vi "ScanCameraFocus.vi"() -> ()   [LabVIEW 2016] (continued)
  out "Match score vs displacement":cluster{dbl[], sgl[]}(graph)={[-2.0, -1.9, -1.8, -1.7, -1.6, -1.5, -1.4, -1.2999999999999998, -1.2, -1.1, -1.0, -0.8999999999999999, -0.7999999999999998, -0.7, -0.5999999999999999, -0.5, -0.3999999999999999, -0.2999999999999998, -0.19999999999999996, -0.09999999999999987, 0.0, 0.10000000000000009, 0.20000000000000018, 0.30000000000000027, 0.40000000000000036, 0.5, 0.6000000000000001, 0.7000000000000002, 0.8000000000000003, 0.9000000000000004, 1.0, 1.1, 1.2000000000000002, 1.3000000000000003, 1.4000000000000004, 1.5, 1.6, 1.7000000000000002, 1.8000000000000003, 1.9000000000000004, 2.0, 2.1000000000000005, 2.2, 2.3, 2.4000000000000004, 2.5, 2.6000000000000005, 2.7, 2.8000000000000007, 2.9000000000000004, 3.0, 3.1000000000000005, 3.2, 3.3000000000000007, 3.4000000000000004, 3.5, 3.6000000000000005, 3.7, 3.8000000000000007, 3.9000000000000004, 4.0, 4.1000000000000005, 4.2, 4.300000000000001, 4.4, 4.5, 4.6000000000000005, 4.7, 4.800000000000001, 4.9, 5.0, 5.1000000000000005, 5.2, 5.300000000000001, 5.4, 5.5, 5.6000000000000005, 5.7, 5.800000000000001, 5.9, 6.0, 6.1, 6.200000000000001, 6.300000000000001, 6.4, 6.5, 6.6, 6.700000000000001, 6.800000000000001, 6.9, 7.0, 7.1, 7.200000000000001, 7.300000000000001, 7.4, 7.5, 7.600000000000001, 7.700000000000001, 7.800000000000001, 7.9, 8.0, 8.100000000000001, 8.200000000000001, 8.3, 8.4, 8.5, 8.600000000000001, 8.700000000000001, 8.8, 8.9, 9.0, 9.100000000000001, 9.200000000000001, 9.3, 9.4, 9.5, 9.600000000000001, 9.700000000000001, 9.8, 9.9, 10.0], [869.16, 870.1541, 871.39026, 872.55273, 873.6957, 875.25287, 876.31866, 877.9247, 879.2218, 880.4835, 881.8531, 883.09845, 884.34955, 886.17163, 887.5967, 888.8688, 890.27716, 892.02856, 893.73047, 895.31525, 896.9751, 898.5983, 900.21747, 902.1295, 904.04614, 905.8335, 907.88635, 910.31226, 912.42053, 914.553, 917.0437, 919.398, 921.9271, 924.781, 928.02673, 931.43286, 934.40283, 937.87115, 941.5338, 945.68744, 948.91864, 952.5989, 956.83673, 960.76074, 964.0517, 967.93036, 970.9311, 973.84906, 976.09045, 976.83105, 978.2025, 977.4351, 976.63086, 976.10803, 972.1438, 968.2719, 965.92584, 962.9048, 957.64667, 955.20544, 950.172, 946.14453, 940.74744, 938.06586, 934.0315, 930.2287, 926.7642, 923.40344, 920.183, 917.18445, 913.9989, 911.6928, 909.2186, 906.7086, 904.7015, 902.61487, 900.4853, 898.55743, 896.5968, 894.7702, 893.13806, 891.5336, 890.0522, 888.5804, 886.85406, 885.3486, 884.04974, 882.66174, 881.2819, 879.8848, 878.6075, 877.4188, 876.1414, 875.2497, 874.0843, 872.85974, 871.7597, 870.1826, 869.6278, 868.561, 867.4404, 866.34564, 865.29114, 864.1999, 863.2289, 862.2323, 861.2315, 859.92535, 859.2958, 858.47675, 857.529, 856.49744, 855.59875, 854.7043, 853.684, 852.79486, 851.9777, 851.04254, 849.966, 848.84424, 848.2957]}
  in  "Match position variation tolerance":sgl=0.25
  out "Z step":dbl=12.0
  out "Image":T1(plugin-control)
  in  "End Z [mm]":dbl=10.0
  in  "Stepsize [mm]":dbl=0.1
  out "Matches (pixel)":T2(array[cluster])=[{"Position"={"x"=1325.479, "y"=883.1293}, "Angle"=0.0, "Scale"=1.0, "Score"=848.2957, "Bounding Box"=[{"x"=657.979, "y"=123.62927}, {"x"=1992.979, "y"=123.62927}, {"x"=1992.979, "y"=1642.6293}, {"x"=657.979, "y"=1642.6293}, {"x"=657.979, "y"=123.62927}]}] {"Bounding Box"."y" format="%.2f"; "Bounding Box"."x" format="%.2f"; "Score" format="%.2f"; "Scale" format="%.2f"; "Angle" format="%.2f"; "Position"."y" format="%.2f"; "Position"."x" format="%.2f"}
  in  "Match parameters":T3={"Number of Matches Requested"=10, "Minimum Match Score"=500.0, "Angle Ranges"=[]}
  in  "Template File Path":path=path "E:/XYZstage+Camera_CollectedImages/12-14-2016/test_sub_highVoltageContact_-23,-32,3.png"
  in  "Axes Speeds [mm/s]":T4={"X Speed"=25.0, "Y Speed"=3.0, "Z Speed"=1.0}
  in  "Initial Location [mm]":T5={"Go to X"=-23.0, "Go to Y"=-32.0, "Go to Z"=-2.0}
  out "Intensity histogram":T6(graph)={"Starting Value"=0.0, "Incremental Value"=1.0, "Histogram"=[77, 310, 1440, 5160, 11707, 21949, 34592, 44040, 61522, 59090, 132881, 181990, 251107, 301599, 277254, 244606, 193626, 125059, 84284, 56323, 35192, 26906, 21597, 17679, 17225, 17011, 10413, 15370, 16520, 15123, 15770, 17568, 16628, 17646, 19451, 17637, 17348, 18783, 16992, 16866, 17857, 16113, 16184, 11662, 16245, 16158, 17494, 16810, 15916, 17260, 16124, 15958, 17021, 16112, 16129, 17034, 15913, 16079, 17096, 15953, 15989, 11536, 16913, 15935, 16847, 16721, 15742, 16537, 17175, 16274, 17105, 17194, 15815, 16580, 16529, 15639, 16024, 15564, 9392, 14100, 14721, 13396, 13560, 14372, 12856, 12836, 13406, 12347, 12091, 12742, 11182, 10888, 11469, 10124, 10025, 10448, 6173, 8856, 9105, 8444, 8061, 8191, 7480, 6963, 7369, 6809, 6453, 6776, 6032, 6067, 6070, 5643, 5289, 3648, 5223, 4907, 4879, 4890, 4361, 4271, 4386, 3978, 4210, 4169, 3975, 3980, 4099, 3655, 3916, 4001, 2490, 3768, 4223, 3979, 4160, 4854, 4741, 5001, 6083, 5999, 6306, 7546, 7880, 8054, 9986, 10168, 9929, 12164, 8022, 12068, 13981, 14724, 14558, 16354, 17360, 16932, 19805, 21358, 21427, 24182, 26203, 25943, 29027, 31067, 29801, 21290, 35655, 35089, 35112, 39088, 37066, 36357, 40319, 38884, 37565, 39954, 37330, 34710, 36959, 34631, 33043, 33818, 30568, 18483, 30035, 26196, 23730, 24039, 20585, 18657, 18863, 16639, 14661, 15185, 12656, 11329, 11618, 9913, 8893, 9157, 5125, 7505, 7274, 6773, 6163, 6256, 5732, 5131, 5344, 4838, 4514, 4667, 4285, 3942, 4133, 3749, 3539, 2267, 3278, 3064, 2952, 2996, 2796, 2575, 2515, 2270, 2133, 2192, 2033, 1877, 1935, 1770, 1663, 1726, 1601, 873, 1561, 1334, 1290, 1371, 1263, 1161, 1232, 1123, 1121, 1221, 1048, 928, 1086, 923, 859, 977, 529, 815, 851, 14587]}
  out "Moving":bool
  out "XYZ Stage Current Position":T7={"X [-750, 750 mm]"=-23.00047348022461, "Y [-150, 30 mm]"=-32.00033050537109, "Z [-50, 50 mm]"=10.000400000000003}
  out "Error report":errorcluster
  in  "Camera Name":refnum<k21>="cam0" caption="IMAQdx Session"
  # "ANALYSIS"
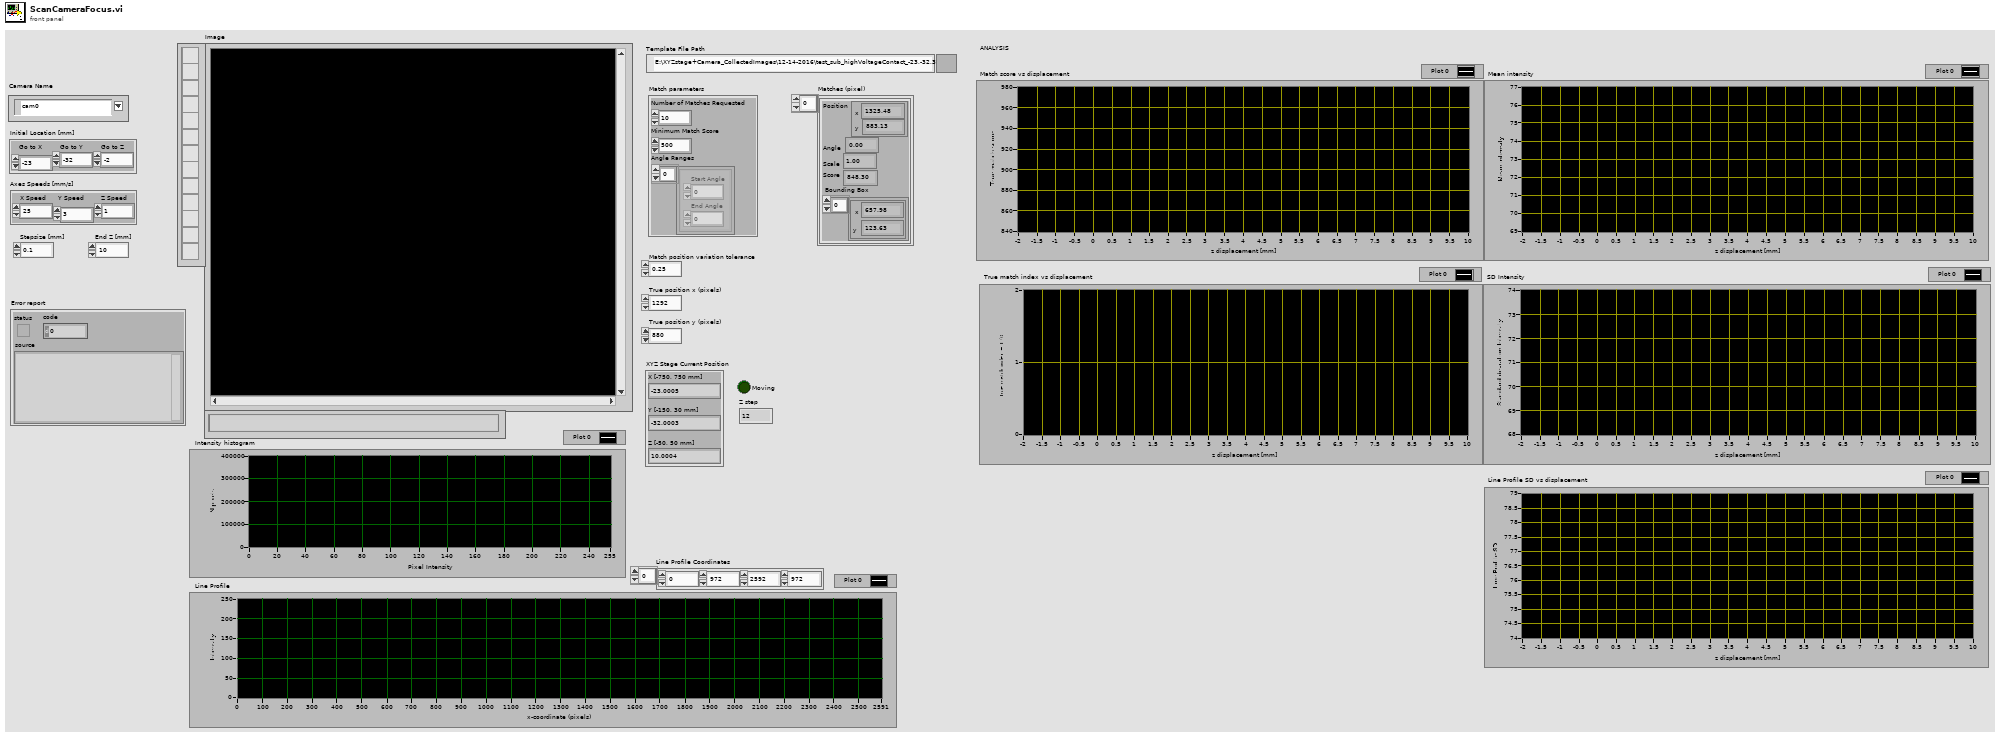
[diagram p1: front panel]
types:
  T1 = typedef "IMAQ Image.ctl" = refnum<image>
  T2 = cluster{"Position":cluster{"x":sgl, "y":sgl}, "Angle":sgl, "Scale":sgl, "Score":sgl, "Bounding Box":cluster{"x":sgl, "y":sgl}[]}[]
  T3 = cluster{"Number of Matches Requested":i32, "Minimum Match Score":sgl, "Angle Ranges":cluster{"Start Angle":sgl, "End Angle":sgl}[]}
  T4 = cluster{"X Speed":dbl, "Y Speed":dbl, "Z Speed":dbl}
  T5 = cluster{"Go to X":dbl, "Go to Y":dbl, "Go to Z":dbl}
  T6 = cluster{"Starting Value":sgl, "Incremental Value":sgl, "Histogram":u32[]}
  T7 = cluster{"X [-750, 750 mm]":dbl, "Y [-150, 30 mm]":dbl, "Z [-50, 50 mm]":dbl}
  T8 = typedef "Image Type" = u32
  T9 = typedef "IMAQdx.ctl" = refnum<k21>
  T10 = cluster{"Final X":dbl, "Final Y":dbl, "Final Z":dbl}
  T11 = cluster{"Min":sgl, "Max":sgl, "Mean":sgl, "Std Dev":sgl, "Count":i32}
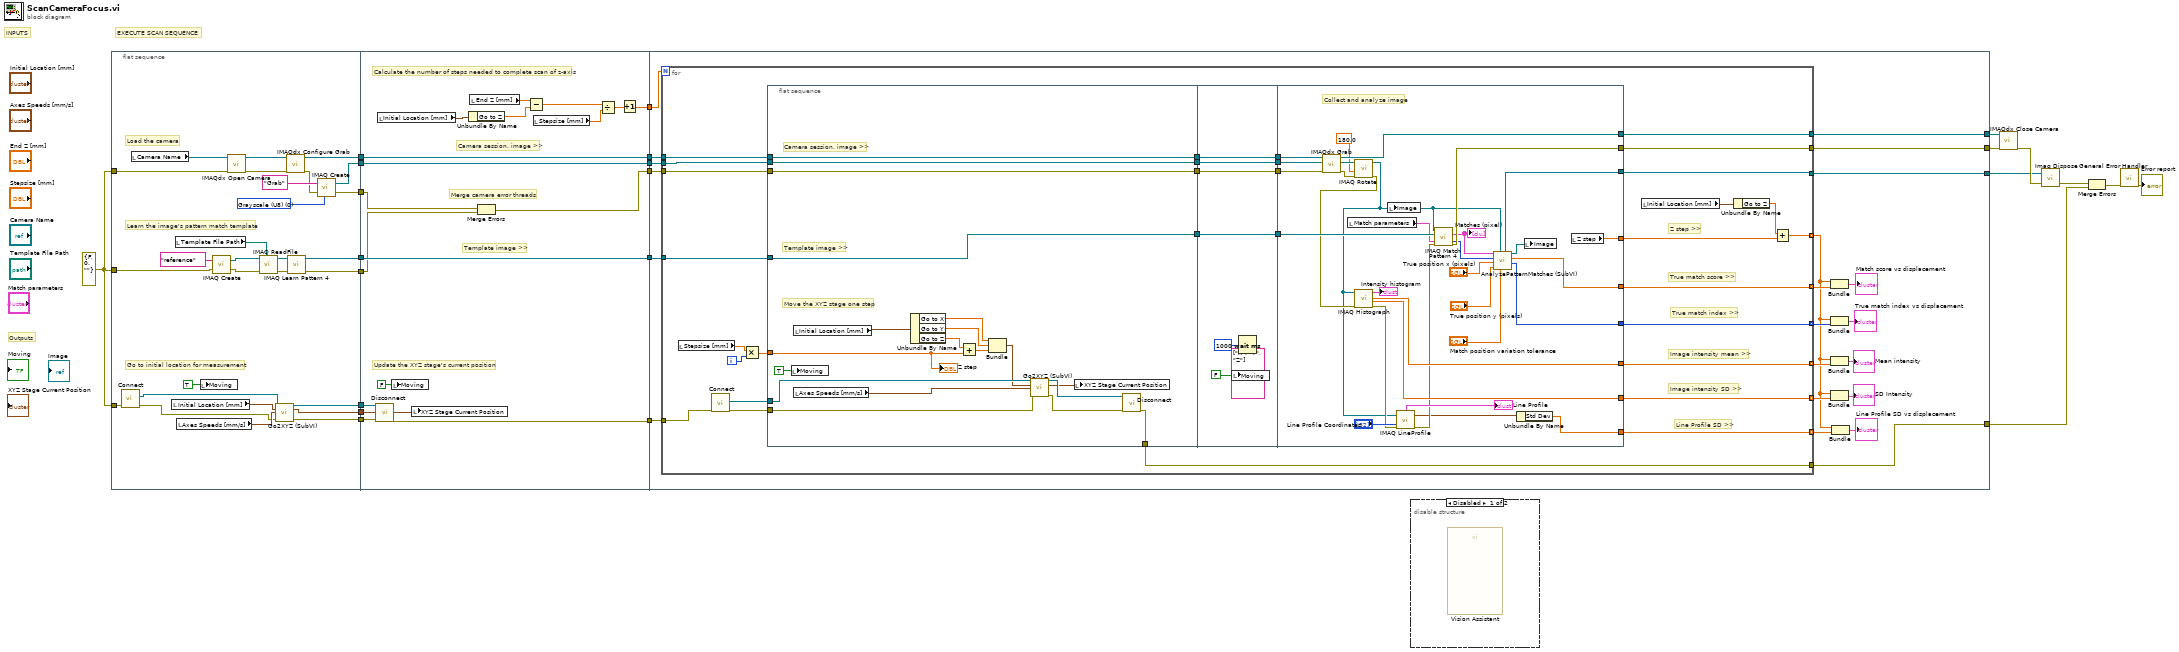
[diagram p0: block diagram]
diagram:
  w2 = errorcluster {"status"=FALSE, "code"=0, "source"=""} ("error in (no error)")
  # "EXECUTE SCAN SEQUENCE"
  # "Outputs"
  # "INPUTS"
  n1 = flat-sequence {
    tunnel: [w51] -> w19
    tunnel: [w50] -> w18
    tunnel: [w45] -> w17
    tunnel: [w34] -> w13
    tunnel: [w30] -> w12
    tunnel: [w29] -> w10
    tunnel: [w28] -> w7
    tunnel: [w27] -> w6
    tunnel: w2 -> [w26]
    tunnel: w2 -> [w25]
    tunnel: w2 -> [w24]
    tunnel: w19 -> [w64]
    tunnel: w18 -> [w63]
    tunnel: w17 -> [w68]
    tunnel: [w52] -> w16
    tunnel: [w62] -> w15
    tunnel: [w60] -> w14
    tunnel: w13 -> [w60]
    tunnel: w12 -> [w59]
    tunnel: [w59] -> w11
    tunnel: w10 -> [w57]
    tunnel: [w55] -> w9
    tunnel: [w58] -> w8
    tunnel: w7 -> [w58]
    tunnel: w6 -> [w56]
    tunnel: w16 -> [w82]
    tunnel: w15 -> [w90]
    tunnel: w14 -> [w89]
    tunnel: w11 -> [w88]
    tunnel: w9 -> [w87]
    tunnel: w8 -> [w86]
    tunnel: [w85] -> w5
    tunnel: [w84] -> w4
    tunnel: [w83] -> w3
    tunnel: [w75] -> w1
    frame #0 {
      w32 = T8 0 items=["Grayscale (U8)", "Grayscale (I16)", "Grayscale (SGL)", "Complex (CSG)", "RGB (U32)", "HSL (U32)", "RGB (U64)", "Grayscale (U16)"] ("Image Type")
      # "Learn the image's pattern match template"
      # "Load the camera"
      # "Go to initial location for measurement"
      n2 = call "Connect.vi"("error in (no error)"=w24) -> ("error out"=w44:errorcluster, "controller"=w46:refnum<k24>)  [unwired: 9 in]
      n3 = local read "Camera Name"() -> (w43:refnum<k21>)
      n4 = local read "Initial Location [mm]"() -> (w47:T5)
      n5 = local read "Template File Path"() -> (w40:path)
      n6 = local read "Axes Speeds [mm/s]"() -> (w48:T4)
      n7 = local write "Moving"(TRUE ("Moving")) -> ()
      n8 = call "IMAQ Create"("Image Name"="reference", "error in (no error)"=w26) -> ("New Image"=w39:T1, "error out"=w38:errorcluster)  [unwired: 3 in]
      n9 = call <vilib>:"IMAQdx Open Camera.vi"("error in"=w25, "Session In"=w43) -> ("error out"=w41:errorcluster, "Session Out"=w42:T9)  [unwired: 1 in, 7 out]
      n10 = call "IMAQ ReadFile"("File Path"=w40, "error in (no error)"=w38, "Image"=w39) -> ("error out"=w35:errorcluster, "Image Out"=w36:T1)  [unwired: 4 in, 3 out]
      n11 = call "Go2XYZ (SubVI).vi"(".NET Refnum in"=w46, "Go to Coordinates"=w47, "Axis Speeds"=w48, "error in (no error)"=w44) -> (".NET Refnum out"=w51:refnum<k24>, "Final Position"=w45:T10, "error out"=w50:errorcluster)  [unwired: 8 in, 1 out]
      n12 = call <vilib>:"IMAQdx Configure Grab.vi"("error in"=w41, "Session In"=w42) -> ("error out"=w31:errorcluster, "Session Out"=w34:T9)  [unwired: 8 out]
      n13 = call "IMAQ Learn Pattern 4"("error in (no error)"=w35, "Image"=w36) -> ("error out"=w27:errorcluster, "Template Image Out"=w28:T1)  [unwired: 7 in, 1 out]
      n14 = call "IMAQ Create"("Image Name"="Grab", "Image Type"=w32, "error in (no error)"=w31) -> ("New Image"=w30:T1, "error out"=w29:errorcluster)  [unwired: 1 in, 1 out]
    }
    frame #1 {
      # "Merge camera error threads"
      # "Camera session, image >>"
      # "Template image >>"
      # "Calculate the number of steps needed to complete scan of z-axis"
      # "Update the XYZ stage's current position"
      n15 = call "Disconnect.vi"("error in (no error)"=w63, "controller"=w64) -> ("error out"=w62:errorcluster)  [unwired: 9 in]
      n16 = local read "Initial Location [mm]"() -> (w67:T5)
      n17 = local write "Moving"(FALSE ("Moving")) -> ()
      n18 = local write "XYZ Stage Current Position"(w68) -> ()
      n19 = Unbundle By Name(w67) -> ("Go to Z"=w66:dbl)
      n20 = local read "End Z [mm]"() -> (w54:dbl)
      n21 = Merge Errors(w57, w56) -> (w55:errorcluster)
      n22 = Subtract(x=w54, y=w66) -> (x-y=w65:dbl)
      n23 = local read "Stepsize [mm]"() -> (w61:dbl)
      n24 = Divide(x=w65, y=w61) -> (x/y=w53:dbl)
      n25 = Increment(x=w53) -> (x+1=w52:dbl)
    }
    frame #2 {
      n26 = for {
        N: w82 -> [_]
        tunnel: w90 -> [w118]
        tunnel: w89 -> [w115]
        tunnel: w88 -> [w114]
        tunnel: w87 -> [w113]
        tunnel: w86 -> [w112]
        tunnel: [w111] -> w85
        tunnel: [w110] -> w84
        tunnel: [w109] -> w83
        tunnel: [w103] -> w71 mode=indexing
        tunnel: [w108] -> w81 mode=indexing
        tunnel: [w107] -> w80 mode=indexing
        tunnel: [w106] -> w79 mode=indexing
        tunnel: [w105] -> w75
        tunnel: [w92] -> w74 mode=indexing
        tunnel: [w91] -> w70 mode=indexing
        i -> [w120]
        (unwired) string[] ["X", "Y", "Z"] ("Axes Names")
        # "Line Profile SD >>"
        # "True match index >>"
        # "Image intensity SD >>"
        # "Image intensity mean >>"
        # "True match score >>"
        # "Z step >>"
        n27 = local read "Stepsize [mm]"() -> (w117:dbl)
        n28 = call "Connect.vi"("error in (no error)"=w118) -> ("error out"=w116:errorcluster, "controller"=w121:refnum<k24>)  [unwired: 9 in]
        n29 = Multiply(x=w117, y=w120) -> (x*y=w119:dbl)
        n30 = flat-sequence {
          tunnel: w121 -> [w140]
          tunnel: w116 -> [w139]
          tunnel: w119 -> [w134]
          tunnel: [w126] -> w100
          tunnel: w115 -> [w126]
          tunnel: w114 -> [w125]
          tunnel: [w125] -> w98
          tunnel: w113 -> [w124]
          tunnel: [w124] -> w96
          tunnel: [w123] -> w94
          tunnel: w112 -> [w123]
          tunnel: [w122] -> w110
          tunnel: w100 -> [w146]
          tunnel: [w146] -> w99
          tunnel: w98 -> [w145]
          tunnel: [w145] -> w97
          tunnel: w96 -> [w144]
          tunnel: [w144] -> w95
          tunnel: w94 -> [w143]
          tunnel: [w143] -> w93
          tunnel: w99 -> [w177]
          tunnel: w97 -> [w176]
          tunnel: w95 -> [w175]
          tunnel: w93 -> [w174]
          tunnel: [w166] -> w111
          tunnel: [w172] -> w109
          tunnel: [w170] -> w101
          tunnel: [w159] -> w108
          tunnel: [w169] -> w107
          tunnel: [w168] -> w106
          tunnel: [w167] -> w105
          tunnel: [w158] -> w92
          tunnel: [w148] -> w91
          frame #0 {
            # "Camera session, image >>"
            # "Template image >>"
            # "Move the XYZ stage one step"
            n31 = local write "Moving"(TRUE ("Moving")) -> ()
            n32 = local read "Initial Location [mm]"() -> (w136:T5)
            n33 = local read "Axes Speeds [mm/s]"() -> (w137:T4)
            n34 = Unbundle By Name(w136) -> ("Go to X"=w131:dbl, "Go to Y"=w132:dbl, "Go to Z"=w135:dbl)
            n35 = Add(x=w135, y=w134) -> (x+y=w133:dbl)
            n36 = Bundle("Go to X"=w131, "Go to Y"=w132, w133) -> (w130:cluster{"Go to X":dbl, "Go to Y":dbl, dbl})  [unwired: 1 in]
            n37 = call "Go2XYZ (SubVI).vi"(".NET Refnum in"=w140, "Go to Coordinates"=w130, "Axis Speeds"=w137, "error in (no error)"=w139) -> (".NET Refnum out"=w129:refnum<k24>, "Final Position"=w127:T10, "error out"=w128:errorcluster)  [unwired: 8 in, 1 out]
            n38 = local write "XYZ Stage Current Position"(w127) -> ()
            n39 = call "Disconnect.vi"("error in (no error)"=w128, "controller"=w129) -> ("error out"=w122:errorcluster)  [unwired: 9 in]
            "Z step" <- w134
          }
          frame #1 {
            n40 = local write "Moving"(FALSE ("Moving")) -> ()
            n41 = Wait (ms)(milliseconds to wait=u32 1000) -> ()  [unwired: 1 out]
          }
          frame #2 {
            # "Collect and analyze image"
            n42 = call <vilib>:"IMAQdx Grab.vi"("error in"=w175, "Image In"=w176, "Session In"=w177) -> ("error out"=w156:errorcluster, "Image Out"=w157:T1, "Session Out"=w172:T9)  [unwired: 1 in, 5 out]
            n43 = local read "Match parameters"() -> (w173:T3)
            n44 = call "IMAQ Rotate"("error in (no error)"=w156, "Angle (degrees)"=sgl 180.0, "Image Src"=w157) -> ("error out"=w155:errorcluster, "Image Dst Out"=w147:T1)  [unwired: 7 in]
            n45 = call "IMAQ Histograph"("error in (no error)"=w155, "Image"=w147) -> ("error out"=w151:errorcluster, "Standard  Deviation"=w168:sgl, "Mean Value"=w169:sgl, "Histogram Graph"=→"Intensity histogram":T6)  [unwired: 6 in]
            n46 = local write "Image"(w147) -> ()
            n47 = call "IMAQ LineProfile"("error in (no error)"=w151, "Line Coordinates"="Line Profile Coordinates", "Image"=w147) -> ("error out"=w150:errorcluster, "Line Graph"=→"Line Profile":cluster{"x0":sgl, "dx":sgl, "Pixels Line":sgl[]}, "Line Information"=w149:T11)  [unwired: 2 in, 1 out]
            n48 = call "IMAQ Match Pattern 4"("Image"=w147, "Template Image"=w174, "Parameters"=w173, "error in (no error)"=w150) -> ("Matches (pixel)"=w163:T2, "Number of Matches"=w164:i32, "error out"=w167:errorcluster)  [unwired: 7 in, 2 out]
            "Matches (pixel)" <- w163
            n49 = call "AnalyzePatternMatches (SubVI).vi"("Match position variation tolerance"="Match position variation tolerance", "Image in"=w147, "true y"="True position y (pixels)", "true x"="True position x (pixels)", "Number of Matches"=w164, "Matches (pixel)"=w163) -> ("True Match Index"=w158:i32, "True Match Score"=w159:sgl, "Display with box"=w165:T1, "Image out"=w166:T1)  [unwired: 2 in]
            n50 = Unbundle By Name(w149) -> ("Std Dev"=w148:sgl)
            n51 = local write "Image"(w165) -> ()
            n52 = local read "Z step"() -> (w170:dbl)
          }
        }
        n53 = local read "Initial Location [mm]"() -> (w104:T5)
        n54 = Unbundle By Name(w104) -> ("Go to Z"=w102:dbl)
        n55 = Add(x=w102, y=w101) -> (x+y=w103:dbl)
      }
      n56 = Bundle(w71, w81) -> (→"Match score vs displacement":cluster{dbl[], sgl[]})  [unwired: 1 in]
      n57 = Bundle(w71, w74) -> (→"True match index vs displacement":cluster{dbl[], i32[]})  [unwired: 1 in]
      n58 = Bundle(w71, w80) -> (→"Mean intensity":cluster{dbl[], sgl[]})  [unwired: 1 in]
      n59 = Bundle(w71, w79) -> (→"SD Intensity":cluster{dbl[], sgl[]})  [unwired: 1 in]
      n60 = Bundle(w71, w70) -> (→"Line Profile SD vs displacement":cluster{dbl[], sgl[]})  [unwired: 1 in]
    }
  }
  n61 = disable-structure shown="Disabled" {
    frame Disabled {
      n62 = call "Vision Assistant"() -> ()  [unwired: 25 in, 3 out]
    }
    frame Enabled {
    }
  }
  n63 = call <vilib>:"IMAQdx Close Camera.vi"("error in"=w1, "Session In"=w3) -> ("error out"=w22:errorcluster)  [unwired: 9 out]
  n64 = call "Imaq Dispose"("Image"=w5, "error in (no error)"=w22) -> ("error out"=w21:errorcluster)  [unwired: 4 in]
  n65 = Merge Errors(w21, w4) -> (w20:errorcluster)
  n66 = call <vilib>:"General Error Handler.vi"("error in (no error)"=w20) -> ("error out"=→"Error report":errorcluster)  [unwired: 2 in, 12 out]
